vi "UHR-Fleezers Control (host) - 12.0.vi"() -> ()   [LabVIEW 2014] (continued)
        n1231 = Divide(x=w1676, y="APD Integration Time (s)") -> (x/y=w1679:dbl)
        n1232 = Multiply(x=2.0, y=w1679) -> (x*y=w1678:dbl)
        n1233 = local write "APD Samples/FIFO Acq."(w1679) -> ()
        n1234 = local write "APD Elements/DMA read"(w1678) -> ()
      }
      event "Number of F/B Scans (AOD)", "Scan Speed (nm/s)", "Scan BD", "Initial D (MHz)", "Step Size (nm)", "Scan Range (nm)", "Wiggle amp 1 (units?)": Value Change {
        w1747 = 123.0  # AOM cal (nm/MHz)
        n1235 = event-data() -> ()  [unwired: 7 out]
        n1236 = local read "BD 1 Frequency 1 (MHz)"() -> (w1730:dbl)
        n1237 = local read "AOM X Cal (nm/MHz)"() -> (w1722:dbl)
        n1238 = local read "BD 2 Frequency 1 (MHz)"() -> (w1736:dbl)
        n1239 = local read "X RF Frequency Limits (MHz)"() -> (w1734:T17)
        n1240 = local read "Y RF Frequency Limits (MHz)"() -> (w1731:T17)
        n1241 = Negate(x="Scan Range (nm)") -> (-x=w1700:dbl)
        n1242 = Divide(x=w1700, y=w1722) -> (x/y=w1704:dbl)
        n1243 = Select(t=w1734, s="Scan BD", f=w1731) -> (s? t:f=w1733:T17)
        n1244 = Select(t=w1730, s="Scan BD", f=w1736) -> (s? t:f=w1735:dbl)
        n1245 = Unbundle By Name(w1733) -> ("Maximum"=w1742:dbl, "Minimum"=w1741:dbl)
        n1246 = Add(x=w1704, y=w1735) -> (x+y=w1739:dbl)
        n1247 = Divide(x=w1700, y="Step Size (nm)") -> (x/y=w1719:dbl)
        n1248 = Divide(x="Step Size (nm)", y=w1722) -> (x/y=w1728:dbl)
        n1249 = Absolute Value(x=w1719) -> (abs(x)=w1703:dbl)
        n1250 = Sign(1:w1700) -> (0:w1701:dbl)
        n1251 = In Range and Coerce(upper limit=w1742, x=w1739, lower limit=w1741) -> (coerced(x)=w1738:dbl, In Range?=w1740:bool)
        n1252 = To Unsigned Quad Integer(1:w1703) -> (0:w1718:u64)
        "Scan steps (AOD)" <- w1718
        n1253 = call "IR AOM freq to word.vi"("Frequency In (MHz)"=w1728) -> ("Frequency Word Out (double)"=w1725:dbl)
        n1254 = Multiply(x=w1701, y=w1725) -> (x*y=w1702:dbl)
        n1255 = Subtract(x=w1739, y=w1738) -> (x-y=w1737:dbl)
        n1256 = To Quad Integer(1:w1702) -> (0:w1724:i64)
        "Incr. int (AOD)" <- w1724
        n1257 = Subtract(x=w1704, y=w1737) -> (x-y=w1723:dbl)
        "Scan Range (MHz)" <- w1723
        n1258 = Select(t=w1704, s=w1740, f=w1723) -> (s? t:f=w1743:dbl)
        n1259 = Multiply(x=w1723, y=w1722) -> (x*y=w1721:dbl)
        n1260 = Decrement(x=w1718) -> (x-1=w1771:u64)
        n1261 = Negate(x=w1721) -> (-x=w1717:dbl)
        n1262 = local write "Scan Range (nm)"(w1717) -> ()
        n1263 = Divide(x=w1743, y=w1771) -> (x/y=w1727:dbl)
        "Scan Increment (MHz)" <- w1727
        n1264 = call "IR AOM freq to word.vi"("Frequency In (MHz)"=w1727) -> ("Frequency Word Out (double)"=w1726:dbl)
        n1265 = Divide(x="Step Size (nm)", y="Scan Speed (nm/s)") -> (x/y=w1714:dbl)
        n1266 = To Quad Integer(1:w1726) -> ()  [unwired: 1 out]
        n1267 = local read "Number Interlace Sets"() -> (w1698:u8)
        n1268 = local read "AI Count (ticks)"() -> (w1699:u32)
        n1269 = local read "Total Counts (ticks)"() -> (w1697:u32)
        n1270 = local read "# Samples/trap"() -> (w1729:u32)
        n1271 = Multiply(x=w1699, y=w1698) -> (x*y=w1696:u32)
        n1272 = Divide(x=w1697, y=w1696) -> (x/y=w1695:dbl)
        n1273 = Select(t=w1730, s="Scan BD", f=w1736) -> (s? t:f=w1768:dbl)
        "Initial freq. (MHz)" <- w1768
        n1274 = Add(x=w1743, y=w1768) -> (x+y=→"Final freq. (MHz)":dbl)
        n1275 = Divide(x=w1697, y=40000000.0) -> (x/y=w1713:dbl)
        n1276 = Divide(x=w1714, y=w1713) -> (x/y=w1712:dbl)
        n1277 = To Unsigned Quad Integer(1:w1712) -> (0:w1687:u64)
        n1278 = Quotient & Remainder(x=w1687, y=u64 2) -> (x-y*floor(x/y)=w1691:u64)  [unwired: 1 out]
        n1279 = Equal?(x=w1691, y=u64 0) -> (x = y?=w1689:bool)
        n1280 = Decrement(x=w1687) -> (x-1=w1688:u64)
        n1281 = Select(t=w1687, s=w1689, f=w1688) -> (s? t:f=w1686:u64)
        "Cycles/step (AOD)" <- w1686
        n1282 = xnode "Read/Write Control"("FPGA VI Reference In"=w1779, "error in"=w1778, "Scan steps"=w1718, "Number of scans"="Number of F/B Scans (AOD)", "Cycles per step"=w1686, "Scan freq.  increment"=w1724, "Scan BD"="Scan BD") -> ("error out"=w1777:errorcluster)  [unwired: 1 out]
        n1283 = Multiply(x=w1718, y=w1686) -> (x*y=w1772:u64)
        n1284 = Multiply(x=w1772, y=u64 2) -> (x*y=w1694:u64)
        n1285 = Multiply(x=w1695, y=w1694) -> (x*y=w1693:dbl)
        "Data points/scan (f/b)" <- w1693
        n1286 = Multiply(x=w1693, y="Number of F/B Scans (AOD)") -> (x*y=w1775:dbl)
        "Data points/scans" <- w1775
        n1287 = Divide(x=w1775, y=w1729) -> (x/y=→"N sets should be saved":dbl)
        n1288 = Multiply(x=w1772, y=w1713) -> (x*y=w1711:dbl)
        "Time/Scan (s) (AOD)" <- w1711
        n1289 = Select(t=w1743, s="Scan BD", f=0.0) -> (s? t:f=w1769:dbl)
        n1290 = Select(t=0.0, s="Scan BD", f=w1743) -> (s? t:f=w1765:dbl)
        n1291 = local read "BD 2 Frequency 2 (MHz)"() -> (w1761:dbl)
        n1292 = local read "BD 1 Frequency 2 (MHz)"() -> (w1764:dbl)
        n1293 = Add(x=w1765, y=w1736) -> (x+y=w1762:dbl)
        n1294 = Add(x=w1730, y=w1769) -> (x+y=w1763:dbl)
        n1295 = Multiply(x=w1711, y=2.0) -> (x*y=w1710:dbl)
        n1296 = Multiply(x=w1710, y="Number of F/B Scans (AOD)") -> (x*y=w1707:dbl)
        n1297 = Divide(x=w1707, y=60.0) -> (x/y=→"Time to Finish All (min)":dbl)
        n1298 = Add(x="Trap 2 Bead Size (nm)", y="Trap 1 Bead Size (nm)") -> (x+y=w1751:dbl)
        n1299 = Divide(x=w1751, y=2.0) -> (x/y=w1745:dbl)
        n1300 = Subtract(x=w1762, y=w1761) -> (x-y=w1759:dbl)
        n1301 = Subtract(x=w1763, y=w1764) -> (x-y=w1760:dbl)
        n1302 = local read "Initial D (MHz)"() -> (w1748:dbl)
        n1303 = Square(x=w1759) -> (x^2=w1758:dbl)
        n1304 = Square(x=w1760) -> (x^2=w1757:dbl)
        n1305 = Add(x=w1757, y=w1758) -> (x+y=w1756:dbl)
        n1306 = Square Root(x=w1756) -> (sqrt(x)=w1755:dbl)
        "Final D (MHz)" <- w1755
        n1307 = Multiply(x=w1747, y=w1755) -> (x*y=w1754:dbl)
        n1308 = Multiply(x=w1748, y=w1747) -> (x*y=w1746:dbl)
        n1309 = Subtract(x=w1746, y=w1745) -> (x-y=→"Initial sep (nm)":dbl)
        n1310 = Subtract(x=w1754, y=w1745) -> (x-y=→"Final sep (nm)":dbl)
      }
      event "Freq or Amp switch first", "Swap F1 and F2", "Freq switch delay", "Amp switch delay": Value Change {
        n1311 = event-data() -> ()  [unwired: 7 out]
        n1312 = local read "Freq or Amp switch first"() -> (w1780:bool)
        n1313 = local read "Amp switch delay"() -> (w1781:u16)
        n1314 = local read "Freq switch delay"() -> (w1783:u16)
        n1315 = local read "Swap F1 and F2"() -> (w1782:bool)
        n1316 = xnode "Read/Write Control"("FPGA VI Reference In"=w1786, "error in"=w1785, "Freq switch delay"=w1783, "Swap F1 and F2"=w1782, "Amp switch delay"=w1781, "Freq or Amp switch first"=w1780) -> ("error out"=w1784:errorcluster)  [unwired: 1 out]
      }
      event "Scan steps (MCL)", "Number of scans (MCL)", "Scan Range (V)\n(of steps)", "2D or 1D Scan", "N APD Samp/step", "Fast Scan Dir", "Continuous MCL Scanning", "Scan lines (y)": Value Change {
        w1788 = 32767.0 ("y")
        n1317 = event-data() -> ()  [unwired: 7 out]
        n1318 = Select(t="Scan lines (y)", s="2D or 1D Scan", f="Number of scans (MCL)") -> (s? t:f=w1793:u64)
        n1319 = Decrement(x="Scan steps (MCL)") -> (x-1=w1809:u64)
        n1320 = Divide(x="Scan Range (V)\n(of steps)", y=w1809) -> (x/y=w1808:dbl)
        "Desired Scan Incr (V)" <- w1808
        n1321 = local read "APD Integration Time (s)"() -> (w1801:dbl)
        n1322 = Multiply(x=w1808, y=w1788) -> (x*y=w1817:dbl)
        n1323 = Divide(x=w1817, y=10.0) -> (x/y=w1807:dbl)
        "Desired incr (int)" <- w1807
        n1324 = local read "Update Count (MCL)"() -> (w1813:u32)
        n1325 = Round Toward -Infinity(1:w1807) -> (0:w1816:dbl)
        n1326 = To Word Integer(number=w1816) -> (16bit integer=w1791:i16)
        "Actual Incr. int (MCL)" <- w1791
        n1327 = Multiply(x=w1801, y=40000000.0) -> (x*y=w1814:dbl)
        n1328 = Divide(x=w1814, y=w1813) -> (x/y=w1812:dbl)
        n1329 = Multiply(x=i16 10, y=w1791) -> (x*y=w1789:i16)
        n1330 = Multiply(x="N APD Samp/step", y=w1812) -> (x*y=w1811:dbl)
        "Cycles/step (MCL)" <- w1811
        n1331 = Divide(x=w1789, y=w1788) -> (x/y=→"Actual MCL Inc (V)":dbl)
        n1332 = Multiply(x="N APD Samp/step", y="Scan steps (MCL)") -> (x*y=w1803:dbl)
        n1333 = local read "APD Samples/FIFO Acq."() -> (w1800:dbl)
        n1334 = Multiply(x=w1803, y=u64 2) -> (x*y=w1802:dbl)
        "Data points/scan (f+b)" <- w1802
        n1335 = Multiply(x=w1802, y=w1793) -> (x*y=w1820:dbl)
        "Data points/scans (MCL)" <- w1820
        n1336 = Multiply(x=w1801, y=w1802) -> (x*y=w1794:dbl)
        "Time/f+b scan (s) (MCL)" <- w1794
        n1337 = Divide(x=w1820, y=w1800) -> (x/y=→"N sets should be saved (MCL)":dbl)
        n1338 = Multiply(x=w1794, y=w1793) -> (x*y=→"Total Time (s)":dbl)
        n1339 = Not(x="Fast Scan Dir") -> (.not. x?=w1798:bool)
        n1340 = xnode "Read/Write Control"("FPGA VI Reference In"=w1824, "error in"=w1823, "Scan steps (MCL)"="Scan steps (MCL)", "Number of scans (MCL)"=w1793, "Cycles per step (MCL)"=w1811, "Scan freq.  increment (MCL)"=w1791, "1D or 2D Scan?"="2D or 1D Scan", "MCL Scan Axis"=w1798, "Cont. Scan (MCL)"="Continuous MCL Scanning") -> ("error out"=w1822:errorcluster)  [unwired: 1 out]
      }
      event "Read Cal": Value Change {
        w1826 = 1000.0 ("y")
        n1341 = event-data() -> ()  [unwired: 7 out]
        n1342 = local read "Save file name"() -> (w1851:path)
        n1343 = local write "Read Cal"(FALSE ("Read Cal")) -> ()
        n1344 = Strip Path(path=w1851) -> (stripped path=w1850:path)  [unwired: 1 out]
        n1345 = Path To String(path=w1850) -> (string=w1849:string)
        n1346 = Concatenate Strings(w1849, "\\current.cal" ("string")) -> (w1847:string)
        n1347 = String To Path(string=w1847) -> (path=w1846:path)
        n1348 = Open/Create/Replace File(file path (use dialog)=w1846, operation (0:open)=T30."open", access (0:read/write)=enum16{"read/write", "read-only", "write-only"}."read-only") -> (refnum out=w1854:refnum<file>, error out=w1840:errorcluster)  [unwired: 1 in, 3 out]
        n1349 = Deny Access(4:w1840, 7:w1854) -> (0:w1839:errorcluster, 3:w1845:refnum<file>)  [unwired: 1 out]
        n1350 = Read from Binary File(5:0.0, 8:w1839, 9:T29."big-endian, network order" ("byte order (0:big-endian, network order)"), 10:-1 ("count (1)"), 11:w1845) -> (0:w1838:errorcluster, 2:w1836:dbl[], 3:w1841:refnum<file>)  [unwired: 2 out]
        n1351 = Array To Cluster(array=w1836) -> (cluster=w1835:T32)
        n1352 = Unbundle(w1835) -> ("[0]"=w1834:dbl, "[1]"=w1833:dbl, "[2]"=w1832:dbl, "[3]"=w1831:dbl, "[4]"=w1830:dbl, "[5]"=w1829:dbl)
        n1353 = Close File(refnum=w1841, error in=w1838) -> (error out=→"Read cal error":errorcluster)  [unwired: 1 out]
        n1354 = Multiply(x=w1829, y=w1826) -> (x*y=w1827:dbl)
        n1355 = local write "T2 k_x (pN/nm)"(w1831) -> ()
        n1356 = local write "T1 k_x (pN/nm)"(w1832) -> ()
        n1357 = local write "T1 a_x (nm/V)"(w1834) -> ()
        n1358 = local write "T2 a_x (nm/V)"(w1833) -> ()
        n1359 = Multiply(x=w1830, y=w1826) -> (x*y=w1828:dbl)
        n1360 = local write "T1 offset_x (mV)"(w1828) -> ()
        n1361 = local write "T2 offset_x (mV)"(w1827) -> ()
      }
      event "Read FX file": Value Change {
        n1362 = event-data() -> ()  [unwired: 7 out]
        n1363 = local write "Read FX file"(FALSE ("Read residual")) -> ()
        n1364 = local read "Save file name"() -> (w1879:path)
        n1365 = Strip Path(path=w1879) -> (stripped path=w1878:path)  [unwired: 1 out]
        n1366 = Path To String(path=w1878) -> (string=w1877:string)
        n1367 = Concatenate Strings(w1877, "\\current.cal" ("string")) -> (w1875:string)
        n1368 = String To Path(string=w1875) -> (path=w1874:path)
        n1369 = Open/Create/Replace File(file path (use dialog)=w1874, operation (0:open)=T30."open", access (0:read/write)=enum16{"read/write", "read-only", "write-only"}."read-only") -> (refnum out=w1871:refnum<file>, error out=w1868:errorcluster)  [unwired: 3 in, 1 out]
        n1370 = Deny Access(4:w1868, 7:w1871) -> (0:w1867:errorcluster, 3:w1870:refnum<file>)  [unwired: 1 in]
        n1371 = Read from Binary File(5:0.0, 8:w1867, 9:T29."big-endian, network order" ("byte order (0:big-endian, network order)"), 10:-1 ("count"), 11:w1870) -> (0:w1863:errorcluster, 2:w1857:dbl[], 3:w1864:refnum<file>)  [unwired: 1 in, 1 out]
        n1372 = Index Array(array=w1857, index=6) -> (element=→"Bad fit error":dbl)
        n1373 = Index Array(array=w1857, index=7) -> (element=→"Fit offset":dbl)
        n1374 = Index Array(array=w1857, index=8) -> (element=→"Hyst. error":dbl)
        n1375 = Close File(refnum=w1864, error in=w1863) -> ()  [unwired: 2 out]
      }
      event "Abort MCL Scan": Value Change {
        n1376 = event-data() -> ()  [unwired: 7 out]
        n1377 = local write "MCL Scanning"(FALSE ("MCL Scanning")) -> ()
        n1378 = xnode "Read/Write Control"("FPGA VI Reference In"=w1884, "error in"=w1883, "Abort scan (MCL)"="Abort MCL Scan") -> ("error out"=w1882:errorcluster)  [unwired: 1 out]
      }
      event "Update Count (MCL)": Value Change {
        n1379 = event-data() -> ()  [unwired: 7 out]
        n1380 = xnode "Read/Write Control"("FPGA VI Reference In"=w1888, "error in"=w1887, "MCL count"="Update Count (MCL)") -> ("error out"=w1886:errorcluster)  [unwired: 1 out]
      }
      event "Phase adjust (MCL)", "+ phase (MCL)", "- phase (MCL)": Value Change {
        n1381 = event-data() -> ()  [unwired: 7 out]
        n1382 = Negate(x="Phase adjust (MCL)") -> (-x=w1897:i16)
        n1383 = Select(t=w1897, s="- phase (MCL)", f="Phase adjust (MCL)") -> (s? t:f=w1895:i16)
        n1384 = Or(x="- phase (MCL)", y="+ phase (MCL)") -> (x .or. y?=w1890:bool)
        n1385 = xnode "Read/Write Control"("FPGA VI Reference In"=w1899, "error in"=w1898, "Phase count adjustment (MCL)"=w1895) -> ("FPGA VI Reference Out"=w1891:T22, "error out"=w1892:errorcluster)
        n1386 = xnode "Read/Write Control"("FPGA VI Reference In"=w1891, "error in"=w1892, "+ phase (MCL)"=w1890) -> ("error out"=w1889:errorcluster)  [unwired: 1 out]
      }
      event "Abort AOD Scan": Value Change {
        n1387 = event-data() -> ()  [unwired: 7 out]
        n1388 = xnode "Read/Write Control"("FPGA VI Reference In"=w1903, "error in"=w1902, "Abort scan"="Abort AOD Scan") -> ("error out"=w1901:errorcluster)  [unwired: 1 out]
      }
      event "Continuous AOD Scanning": Value Change {
        n1389 = event-data() -> ()  [unwired: 7 out]
        n1390 = xnode "Read/Write Control"("FPGA VI Reference In"=w1907, "error in"=w1906, "Cont. Scan"="Continuous AOD Scanning") -> ("error out"=w1905:errorcluster)  [unwired: 1 out]
      }
      event "Index": Value Change {
        n1391 = event-data() -> ()  [unwired: 7 out]
        n1392 = call "Create new save file.vi"("Insert"="", "Ext"=".dat" ("string"), "Index In"="Index") -> ("Path Out"=→"Save file name":path, "Index Out"=w1908:dbl)
        "Save index" <- w1908
        n1393 = local write "Index"(w1908) -> ()
      }
      event "AO1", "AO2": Value Change {
        w1923 = 10.0 ("y")
        w1922 = 32767.0 ("y")
        n1394 = event-data() -> ()  [unwired: 7 out]
        n1395 = local read "AO2"() -> (w1921:dbl)
        n1396 = local read "AO1"() -> (w1918:dbl)
        n1397 = Multiply(x=w1918, y=w1922) -> (x*y=w1917:dbl)
        n1398 = Multiply(x=w1921, y=w1922) -> (x*y=w1920:dbl)
        n1399 = Divide(x=w1917, y=w1923) -> (x/y=w1916:dbl)
        n1400 = Divide(x=w1920, y=w1923) -> (x/y=w1919:dbl)
        n1401 = To Word Integer(number=w1916) -> (16bit integer=w1924:i16)
        n1402 = To Word Integer(number=w1919) -> (16bit integer=w1925:i16)
        n1403 = xnode "Read/Write Control"("FPGA VI Reference In"=w1915, "error in"=w1914, "AO1"=w1924, "AO2"=w1925) -> ("error out"=w1913:errorcluster)  [unwired: 1 out]
      }
      event "Inject Pump 1": Value Change {
        n1404 = event-data() -> ()  [unwired: 7 out]
        n1405 = local read "Use Harvard pumps\nfor beads (else Chemyx)"() -> (w1927:bool)
        n1406 = case shown="True" w1927 {
          tunnel: "Inject Pump 1" -> [w1931 w1969]
          tunnel: w1926 -> [_ w1970]
          frame False {
            n1407 = local read "Pump write delay (ms)"() -> (w1930:dbl)
            n1408 = local read "Chemyx Syringe Pump Serial Port"() -> (w1929:refnum<visa-resource-name>)
            n1409 = case shown="True" w1931 {
              tunnel: w1930 -> [w1937 w1951]
              tunnel: w1929 -> [w1934 w1950]
              frame False {
                n1410 = flat-sequence {
                  tunnel: w1934 -> [w1938]
                  tunnel: [w1938] -> w1935
                  tunnel: w1937 -> [_]
                  tunnel: [w1941] -> w1936
                  tunnel: w1935 -> [w1941]
                  tunnel: w1936 -> [w1942]
                  tunnel: [w1942] -> w1932
                  tunnel: [w1944] -> w1933
                  tunnel: w1932 -> [w1944]
                  tunnel: w1933 -> [w1946]
                  frame #0 {
                    n1411 = call "Write to pump.vi"("string"="enter pump1", "VISA resource name"=w1938) -> ()  [unwired: 1 out]
                  }
                  frame #1 {
                    n1412 = Wait (ms)(milliseconds to wait="Pump pause delay (ms)") -> ()  [unwired: 1 out]
                  }
                  frame #2 {
                    n1413 = call "Write to pump.vi"("string"="stop", "VISA resource name"=w1942) -> ()  [unwired: 1 out]
                  }
                  frame #3 {
                    n1414 = Wait (ms)(milliseconds to wait=u32 500) -> ()  [unwired: 1 out]
                  }
                  frame #4 {
                    n1415 = call "Write to pump.vi"("string"="stop", "VISA resource name"=w1946) -> ()  [unwired: 1 out]
                  }
                }
              }
              frame True {
                n1416 = flat-sequence {
                  tunnel: w1950 -> [w1960]
                  tunnel: w1951 -> [w1955]
                  tunnel: w1951 -> [w1962]
                  tunnel: w1950 -> [w1963]
                  tunnel: [w1963] -> w1948
                  tunnel: [w1965] -> w1949
                  tunnel: w1948 -> [w1965]
                  tunnel: w1949 -> [w1967]
                  frame #0 {
                    n1417 = local read "All Pump Parameters"() -> (w1954:T5)
                    n1418 = Unbundle By Name(w1954) -> ("Pump 1"=w1961:T33)
                    n1419 = call "Set pump parameters.vi"("Pump write delay (ms)"=w1955, "Volume (uL)"="Ch 1 Inject Volume (uL)", "Rate (uL/h)"="Ch 1 Inject Rate (ul/h)", "Units"=4.0, "Pump #"=1.0, "Pump Parameters In"=w1961, "VISA resource name"=w1960) -> ("Pump Parameters Out"=w1953:T33)  [unwired: 3 in]
                    n1420 = Bundle By Name(cluster=w1954, "Pump 1"=w1953) -> (w1952:T5)
                    n1421 = local write "All Pump Parameters"(w1952) -> ()
                  }
                  frame #1 {
                    n1422 = Wait (ms)(milliseconds to wait=w1962) -> ()  [unwired: 1 out]
                  }
                  frame #2 {
                    n1423 = call "Write to pump.vi"("string"="start", "VISA resource name"=w1963) -> ()  [unwired: 1 out]
                  }
                  frame #3 {
                    n1424 = Wait (ms)(milliseconds to wait=u32 500) -> ()  [unwired: 1 out]
                  }
                  frame #4 {
                    n1425 = call "Write to pump.vi"("string"="start", "VISA resource name"=w1967) -> ()  [unwired: 1 out]
                  }
                }
              }
            }
          }
          frame True {
            n1426 = case shown="True" w1969 {
              tunnel: w1970 -> [w1971 w1981]
              frame False {
                n1427 = flat-sequence {
                  tunnel: w1971 -> [w1973]
                  frame #0 {
                    n1428 = local write "Flushing P1"(FALSE ("Flushing P1")) -> ()
                    n1429 = Concatenate Strings("stop" ("string"), "\r") -> (w1975:string)
                    n1430 = VISA Write(VISA resource name=w1973, write buffer=w1975) -> ()  [unwired: 1 in, 3 out]
                  }
                  frame #1 {
                    n1431 = property on="Clear Volume P1" class="Bool (strict)"("Val(Sgnl)"=TRUE ("Value (Signaling)")) -> ()  [unwired: 2 in, 2 out]
                  }
                }
              }
              frame True {
                n1432 = local read "Normal Flow Rate (ul/h) P1"() -> (w1979:dbl)
                n1433 = Number To Decimal String(number=w1979) -> (decimal integer string=w1985:string)  [unwired: 1 in]
                n1434 = Concatenate Strings("irate  " ("string"), w1985, " u/h" ("string"), "\r") -> (w1983:string)
                n1435 = VISA Write(VISA resource name=w1981, write buffer=w1983) -> (VISA resource name out=w1980:refnum<visa-resource-name>)  [unwired: 1 in, 2 out]
                n1436 = Concatenate Strings("irun" ("string"), "\r") -> (w1987:string)
                n1437 = VISA Write(VISA resource name=w1980, write buffer=w1987) -> ()  [unwired: 1 in, 3 out]
              }
            }
          }
        }
      }
      event "Inject Pump 3": Value Change {
        n1438 = event-data() -> ()  [unwired: 7 out]
        n1439 = local read "Use Harvard pumps\nfor beads (else Chemyx)"() -> (w1990:bool)
        n1440 = case shown="True" w1990 {
          tunnel: "Inject Pump 3" -> [w1994 w2033]
          tunnel: w1989 -> [_ w2032]
          frame False {
            n1441 = local read "Pump write delay (ms)"() -> (w1993:dbl)
            n1442 = case shown="True" w1994 {
              tunnel: w1993 -> [w2000 w2014]
              tunnel: "Chemyx Syringe Pump Serial Port" -> [w1997 w2013]
              frame False {
                n1443 = flat-sequence {
                  tunnel: w1997 -> [w2001]
                  tunnel: [w2001] -> w1998
                  tunnel: w2000 -> [_]
                  tunnel: [w2004] -> w1999
                  tunnel: w1998 -> [w2004]
                  tunnel: w1999 -> [w2005]
                  tunnel: [w2005] -> w1995
                  tunnel: [w2007] -> w1996
                  tunnel: w1995 -> [w2007]
                  tunnel: w1996 -> [w2009]
                  frame #0 {
                    n1444 = call "Write to pump.vi"("string"="enter pump3", "VISA resource name"=w2001) -> ()  [unwired: 1 out]
                  }
                  frame #1 {
                    n1445 = local read "Pump pause delay (ms)"() -> (w2003:u32)
                    n1446 = Wait (ms)(milliseconds to wait=w2003) -> ()  [unwired: 1 out]
                  }
                  frame #2 {
                    n1447 = call "Write to pump.vi"("string"="stop", "VISA resource name"=w2005) -> ()  [unwired: 1 out]
                  }
                  frame #3 {
                    n1448 = Wait (ms)(milliseconds to wait=u32 0) -> ()  [unwired: 1 out]
                  }
                  frame #4 {
                    n1449 = call "Write to pump.vi"("string"="stop", "VISA resource name"=w2009) -> ()  [unwired: 1 out]
                  }
                }
              }
              frame True {
                n1450 = flat-sequence {
                  tunnel: w2013 -> [w2023]
                  tunnel: w2014 -> [w2018]
                  tunnel: w2014 -> [w2025]
                  tunnel: w2013 -> [w2026]
                  tunnel: [w2026] -> w2012
                  tunnel: [w2029] -> w2011
                  tunnel: w2012 -> [w2029]
                  tunnel: w2011 -> [w2030]
                  frame #0 {
                    n1451 = local read "All Pump Parameters"() -> (w2017:T5)
                    n1452 = Unbundle By Name(w2017) -> ("Pump 3"=w2024:T33)
                    n1453 = call "Set pump parameters.vi"("Pump write delay (ms)"=w2018, "Volume (uL)"="Ch 3 Inject Volume (uL)", "Rate (uL/h)"="Ch 3 Inject Rate (ul/h)", "Units"=4.0, "Pump #"=3.0, "Pump Parameters In"=w2024, "VISA resource name"=w2023) -> ("Pump Parameters Out"=w2016:T33)  [unwired: 3 in]
                    n1454 = Bundle By Name(cluster=w2017, "Pump 3"=w2016) -> (w2015:T5)
                    n1455 = local write "All Pump Parameters"(w2015) -> ()
                  }
                  frame #1 {
                    n1456 = Wait (ms)(milliseconds to wait=w2025) -> ()  [unwired: 1 out]
                  }
                  frame #2 {
                    n1457 = call "Write to pump.vi"("string"="start", "VISA resource name"=w2026) -> ()  [unwired: 1 out]
                  }
                  frame #3 {
                    n1458 = Wait (ms)(milliseconds to wait=u32 500) -> ()  [unwired: 1 out]
                  }
                  frame #4 {
                    n1459 = call "Write to pump.vi"("string"="start", "VISA resource name"=w2030) -> ()  [unwired: 1 out]
                  }
                }
              }
            }
          }
          frame True {
            n1460 = case shown="True" w2033 {
              tunnel: w2032 -> [w2034 w2041]
              frame False {
                n1461 = flat-sequence {
                  tunnel: w2034 -> [w2036]
                  frame #0 {
                    n1462 = local write "Flushing P3"(FALSE ("Flushing P3")) -> ()
                    n1463 = Concatenate Strings("stop" ("string"), "\r") -> (w2038:string)
                    n1464 = VISA Write(VISA resource name=w2036, write buffer=w2038) -> ()  [unwired: 1 in, 3 out]
                  }
                  frame #1 {
                    n1465 = property on="Clear Volume P3" class="Bool (strict)"("Val(Sgnl)"=TRUE ("Value (Signaling)")) -> ()  [unwired: 2 in, 2 out]
                  }
                }
              }
              frame True {
                n1466 = local read "Normal Flow Rate (ul/h) P3"() -> (w2042:dbl)
                n1467 = Number To Decimal String(number=w2042) -> (decimal integer string=w2048:string)  [unwired: 1 in]
                n1468 = Concatenate Strings("irate  " ("string"), w2048, " u/h" ("string"), "\r") -> (w2046:string)
                n1469 = VISA Write(VISA resource name=w2041, write buffer=w2046) -> (VISA resource name out=w2044:refnum<visa-resource-name>)  [unwired: 1 in, 2 out]
                n1470 = Concatenate Strings("irun" ("string"), "\r") -> (w2050:string)
                n1471 = VISA Write(VISA resource name=w2044, write buffer=w2050) -> ()  [unwired: 1 in, 3 out]
              }
            }
          }
        }
      }
      event "Inject Pump 2": Value Change {
        n1472 = event-data() -> ()  [unwired: 7 out]
        n1473 = local read "Pump write delay (ms)"() -> (w2054:dbl)
        n1474 = local read "Chemyx Syringe Pump Serial Port"() -> (w2052:refnum<visa-resource-name>)
        n1475 = flat-sequence {
          tunnel: w2052 -> [w2067]
          tunnel: w2054 -> [w2063]
          tunnel: "Inject Pump 2" -> [_]
          tunnel: w2054 -> [w2069]
          tunnel: w2052 -> [w2070]
          frame #0 {
            n1476 = local read "All Pump Parameters"() -> (w2062:T5)
            n1477 = Multiply(x=60.0, y="Flush Center Ch Rate (ul/m)") -> (x*y=w2059:dbl)
            n1478 = Unbundle By Name(w2062) -> ("Pump 2"=w2068:T33)
            n1479 = call "Set pump parameters.vi"("Pump write delay (ms)"=w2063, "Volume (uL)"="Flush Center Ch Volume (uL)", "Rate (uL/h)"=w2059, "Units"=3.0, "Pump #"=2.0, "Pump Parameters In"=w2068, "VISA resource name"=w2067) -> ("Pump Parameters Out"=w2061:T33)  [unwired: 3 in]
            n1480 = Bundle By Name(cluster=w2062, "Pump 2"=w2061) -> (w2060:T5)
            n1481 = Add(x="Flush Center Ch Volume (uL)", y="Total Volume\nFlushed (uL)") -> (x+y=w2056:dbl)
            n1482 = local write "All Pump Parameters"(w2060) -> ()
            n1483 = local write "Total Volume\nFlushed (uL)"(w2056) -> ()
          }
          frame #1 {
            n1484 = Wait (ms)(milliseconds to wait=w2069) -> ()  [unwired: 1 out]
          }
          frame #2 {
            n1485 = call "Write to pump.vi"("string"="start", "VISA resource name"=w2070) -> ()  [unwired: 1 out]
          }
        }
      }
      event "Sample Channel\nFlow": Value Change {
        n1486 = event-data() -> ()  [unwired: 7 out]
        n1487 = case shown="True" "Sample Channel\nFlow" {
          tunnel: w2073 -> [w2074 w2080]
          frame False {
            n1488 = flat-sequence {
              tunnel: w2074 -> [w2076]
              frame #0 {
                n1489 = local write "Flushing samp"(FALSE ("Flushing samp")) -> ()
                n1490 = Concatenate Strings("stop" ("string"), "\r") -> (w2079:string)
                n1491 = VISA Write(VISA resource name=w2076, write buffer=w2079) -> ()  [unwired: 1 in, 3 out]
              }
            }
          }
          frame True {
            n1492 = local read "Normal Flow rate (mL/h)"() -> (w2090:dbl)
            n1493 = Number To Decimal String(number=w2090) -> (decimal integer string=w2089:string)  [unwired: 1 in]
            n1494 = Concatenate Strings("irate " ("string"), w2089, " u/h" ("string"), "\r") -> (w2085:string)
            n1495 = VISA Write(VISA resource name=w2080, write buffer=w2085) -> (VISA resource name out=w2084:refnum<visa-resource-name>)  [unwired: 1 in, 2 out]
            n1496 = Concatenate Strings("irun" ("string"), "\r") -> (w2081:string)
            n1497 = VISA Write(VISA resource name=w2084, write buffer=w2081) -> ()  [unwired: 1 in, 3 out]
          }
        }
      }
      event "Start Flow": Value Change {
        n1498 = event-data() -> ()  [unwired: 7 out]
        n1499 = local write "Sample Channel\nFlow"(TRUE ("Sample Channel\nFlow")) -> ()
        n1500 = local write "Start Flow"(FALSE ("Start Flow")) -> ()
        n1501 = Concatenate Strings("irun" ("string"), "\r") -> (w2095:string)
        n1502 = VISA Write(VISA resource name=w2091, write buffer=w2095) -> ()  [unwired: 1 in, 3 out]
      }
      event "Stop Flow": Value Change {
        w2097 = FALSE ("Stop Flow")
        n1503 = event-data() -> ()  [unwired: 7 out]
        n1504 = local write "Stop Flow"(w2097) -> ()
        n1505 = local write "Sample Channel\nFlow"(w2097) -> ()
        n1506 = Concatenate Strings("stop" ("string"), "\r") -> (w2100:string)
        n1507 = VISA Write(VISA resource name=w2098, write buffer=w2100) -> ()  [unwired: 1 in, 3 out]
      }
      event "Normal Flow rate (mL/h)": Value Change {
        n1508 = event-data() -> ()  [unwired: 7 out]
        n1509 = Number To Decimal String(number="Normal Flow rate (mL/h)") -> (decimal integer string=w2107:string)  [unwired: 1 in]
        n1510 = Concatenate Strings("irate  " ("string"), w2107, " u/h" ("string"), "\r") -> (w2106:string)
        n1511 = VISA Write(VISA resource name=w2103, write buffer=w2106) -> ()  [unwired: 1 in, 3 out]
      }
      event "Flush Sample": Value Change {
        n1512 = event-data() -> ()  [unwired: 7 out]
        n1513 = flat-sequence {
          tunnel: w2109 -> [w2137]
          frame #0 {
            # "set parameters (rate, volume) for flush, clear volume"
            n1514 = Number To Decimal String(number="Flush rate (mL/m)") -> (decimal integer string=w2133:string)  [unwired: 1 in]
            n1515 = local write "Sample Channel\nFlow"(TRUE ("Sample Channel\nFlow")) -> ()
            n1516 = Concatenate Strings("irate  " ("string"), w2133, " u/m" ("string"), "\r") -> (w2135:string)
            n1517 = VISA Write(VISA resource name=w2137, write buffer=w2135) -> (VISA resource name out=w2131:refnum<visa-resource-name>)  [unwired: 1 in, 2 out]
            n1518 = Number To Decimal String(number="Flush volume (mL)") -> (decimal integer string=w2122:string)  [unwired: 1 in]
            n1519 = Reciprocal(x="Flush rate (mL/m)") -> (1/x=w2116:dbl)
            n1520 = Concatenate Strings("tvolume  " ("string"), w2122, " u" ("string"), "\r") -> (w2120:string)
            n1521 = Multiply(x=w2116, y="Flush volume (mL)") -> (x*y=w2114:dbl)
            n1522 = VISA Write(VISA resource name=w2131, write buffer=w2120) -> (VISA resource name out=w2119:refnum<visa-resource-name>)  [unwired: 1 in, 2 out]
            n1523 = Multiply(x=w2114, y=60.0) -> (x*y=→"Samp Flush Time (s)":dbl)
            n1524 = Concatenate Strings("cvolume" ("string"), "\r") -> (w2118:string)
            n1525 = VISA Write(VISA resource name=w2119, write buffer=w2118) -> (VISA resource name out=w2129:refnum<visa-resource-name>)  [unwired: 1 in, 2 out]
            n1526 = Concatenate Strings("irun" ("string"), "\r") -> (w2127:string)
            n1527 = VISA Write(VISA resource name=w2129, write buffer=w2127) -> ()  [unwired: 1 in, 3 out]
          }
          frame #1 {
            "Flushing samp" <- TRUE ("Boolean")
          }
        }
      }
      event "Flush Pump 3": Value Change {
        n1528 = event-data() -> ()  [unwired: 7 out]
        n1529 = flat-sequence {
          tunnel: w2139 -> [w2142]
          frame #0 {
            # "set paramaters (rate, volume) for flush, clear volume"
            n1530 = Number To Decimal String(number="Flush rate (uL/m) P3") -> (decimal integer string=w2164:string)  [unwired: 1 in]
            n1531 = local write "Inject Pump 3"(TRUE ("Inject Pump 3")) -> ()
            n1532 = Concatenate Strings("irate  " ("string"), w2164, " u/m" ("string"), "\r") -> (w2166:string)
            n1533 = VISA Write(VISA resource name=w2142, write buffer=w2166) -> (VISA resource name out=w2162:refnum<visa-resource-name>)  [unwired: 1 in, 2 out]
            n1534 = Reciprocal(x="Flush rate (uL/m) P3") -> (1/x=w2146:dbl)
            n1535 = Number To Decimal String(number="Volume (uL) P3") -> (decimal integer string=w2153:string)  [unwired: 1 in]
            n1536 = Multiply(x="Volume (uL) P3", y=w2146) -> (x*y=w2145:dbl)
            n1537 = Concatenate Strings("tvolume  " ("string"), w2153, " u" ("string"), "\r") -> (w2151:string)
            n1538 = Multiply(x=w2145, y=60.0) -> (x*y=→"HP3 Flush Time (s)":dbl)
            n1539 = VISA Write(VISA resource name=w2162, write buffer=w2151) -> (VISA resource name out=w2150:refnum<visa-resource-name>)  [unwired: 1 in, 2 out]
            n1540 = Concatenate Strings("cvolume" ("string"), "\r") -> (w2149:string)
            n1541 = VISA Write(VISA resource name=w2150, write buffer=w2149) -> (VISA resource name out=w2160:refnum<visa-resource-name>)  [unwired: 1 in, 2 out]
            n1542 = Concatenate Strings("irun" ("string"), "\r") -> (w2158:string)
            n1543 = VISA Write(VISA resource name=w2160, write buffer=w2158) -> ()  [unwired: 1 in, 3 out]
          }
          frame #1 {
            "Flushing P3" <- TRUE ("Flushing P3")
          }
        }
      }
      event "Flush Pump 1": Value Change {
        n1544 = event-data() -> ()  [unwired: 7 out]
        n1545 = flat-sequence {
          tunnel: [w2180] -> w2170
          tunnel: w2169 -> [w2173]
          tunnel: w2170 -> [_]
          frame #0 {
            # "set paramaters (rate, volume) for flush, clear volume"
            n1546 = local write "Inject Pump 1"(TRUE ("Inject Pump 1")) -> ()
            n1547 = Number To Decimal String(number="Flush rate (uL/m) P1") -> (decimal integer string=w2196:string)  [unwired: 1 in]
            n1548 = Concatenate Strings("irate  " ("string"), w2196, " u/m" ("string"), "\r") -> (w2198:string)
            n1549 = VISA Write(VISA resource name=w2173, write buffer=w2198) -> (VISA resource name out=w2194:refnum<visa-resource-name>)  [unwired: 1 in, 2 out]
            n1550 = Reciprocal(x="Flush rate (uL/m) P1") -> (1/x=w2177:dbl)
            n1551 = Number To Decimal String(number="Volume (uL) P1") -> (decimal integer string=w2185:string)  [unwired: 1 in]
            n1552 = Multiply(x="Volume (uL) P1", y=w2177) -> (x*y=w2176:dbl)
            n1553 = Concatenate Strings("tvolume  " ("string"), w2185, " u" ("string"), "\r") -> (w2183:string)
            n1554 = Multiply(x=w2176, y=60.0) -> (x*y=→"HP1 Flush Time (s)":dbl)
            n1555 = VISA Write(VISA resource name=w2194, write buffer=w2183) -> (VISA resource name out=w2182:refnum<visa-resource-name>)  [unwired: 1 in, 2 out]
            n1556 = Concatenate Strings("cvolume" ("string"), "\r") -> (w2181:string)
            n1557 = VISA Write(VISA resource name=w2182, write buffer=w2181) -> (VISA resource name out=w2192:refnum<visa-resource-name>)  [unwired: 1 in, 2 out]
            n1558 = Concatenate Strings("irun" ("string"), "\r") -> (w2190:string)
            n1559 = VISA Write(VISA resource name=w2192, write buffer=w2190) -> (VISA resource name out=w2180:refnum<visa-resource-name>)  [unwired: 1 in, 2 out]
          }
          frame #1 {
            "Flushing P1" <- TRUE ("Flushing P3")
          }
        }
      }
      event "Clear Volume": Value Change {
        n1560 = event-data() -> ()  [unwired: 7 out]
        n1561 = Number To Decimal String(number="Normal volume (mL)") -> (decimal integer string=w2205:string)  [unwired: 1 in]
        n1562 = Concatenate Strings("tvolume " ("string"), w2205, " u" ("string"), "\r") -> (w2202:string)
        n1563 = VISA Write(VISA resource name=w2208, write buffer=w2202) -> (VISA resource name out=w2201:refnum<visa-resource-name>)  [unwired: 1 in, 2 out]
        n1564 = local write "Clear Volume"(FALSE ("Clear Volume")) -> ()
        n1565 = Concatenate Strings("cvolume" ("string"), "\r") -> (w2210:string)
        n1566 = VISA Write(VISA resource name=w2201, write buffer=w2210) -> ()  [unwired: 1 in, 3 out]
      }
      event "Clear Volume P3": Value Change {
        n1567 = event-data() -> ()  [unwired: 7 out]
        n1568 = Concatenate Strings("cvolume" ("string"), "\r") -> (w2216:string)
        n1569 = VISA Write(VISA resource name=w2215, write buffer=w2216) -> ()  [unwired: 1 in, 3 out]
        n1570 = local write "Clear Volume P3"(FALSE ("Clear Volume P3")) -> ()
      }
      event "Clear Volume P1": Value Change {
        n1571 = event-data() -> ()  [unwired: 7 out]
        n1572 = Concatenate Strings("cvolume" ("string"), "\r") -> (w2221:string)
        n1573 = local write "Clear Volume P1"(FALSE ("Clear Volume P1")) -> ()
        n1574 = VISA Write(VISA resource name=w2220, write buffer=w2221) -> ()  [unwired: 1 in, 3 out]
      }
      event "Display On P3": Value Change {
        n1575 = event-data() -> ()  [unwired: 7 out]
        n1576 = Select(t="dim 100", s="Display On P3", f="dim 0") -> (s? t:f=w2227:string)
        n1577 = Concatenate Strings(w2227, "\r") -> (w2229:string)
        n1578 = VISA Write(VISA resource name=w2224, write buffer=w2229) -> ()  [unwired: 1 in, 3 out]
      }
      event "Display On P1": Value Change {
        n1579 = event-data() -> ()  [unwired: 7 out]
        n1580 = Select(t="dim 100", s="Display On P1", f="dim 0") -> (s? t:f=w2234:string)
        n1581 = Concatenate Strings(w2234, "\r") -> (w2236:string)
        n1582 = VISA Write(VISA resource name=w2231, write buffer=w2236) -> ()  [unwired: 1 in, 3 out]
      }
      event "Retract Pump 3": Value Change {
        n1583 = event-data() -> ()  [unwired: 7 out]
        n1584 = local write "Retract Pump 3"(FALSE ("Retract Pump 3")) -> ()
        n1585 = case shown="True" "Retract Pump 3" {
          tunnel: w2238 -> [_ w2241]
          frame False {
          }
          frame True {
            n1586 = Number To Decimal String(number="Retract Rate (mL/m)") -> (decimal integer string=w2259:string)  [unwired: 1 in]
            n1587 = Concatenate Strings("wrate  " ("string"), w2259, " u/m" ("string"), "\r") -> (w2261:string)
            n1588 = VISA Write(VISA resource name=w2241, write buffer=w2261) -> (VISA resource name out=w2252:refnum<visa-resource-name>)  [unwired: 1 in, 2 out]
            n1589 = Number To Decimal String(number="Retract Vol 3 (uL)") -> (decimal integer string=w2254:string)  [unwired: 1 in]
            n1590 = Concatenate Strings("tvolume  " ("string"), w2254, " u" ("string"), "\r") -> (w2251:string)
            n1591 = VISA Write(VISA resource name=w2252, write buffer=w2251) -> (VISA resource name out=w2247:refnum<visa-resource-name>)  [unwired: 1 in, 2 out]
            n1592 = Concatenate Strings("cvolume" ("string"), "\r") -> (w2248:string)
            n1593 = VISA Write(VISA resource name=w2247, write buffer=w2248) -> (VISA resource name out=w2242:refnum<visa-resource-name>)  [unwired: 1 in, 2 out]
            n1594 = Concatenate Strings("wrun" ("string"), "\r") -> (w2243:string)
            n1595 = VISA Write(VISA resource name=w2242, write buffer=w2243) -> ()  [unwired: 1 in, 3 out]
          }
        }
      }
      event "Retract Pump 1": Value Change {
        n1596 = event-data() -> ()  [unwired: 7 out]
        n1597 = local write "Retract Pump 1"(FALSE ("Retract Pump 1")) -> ()
        n1598 = case shown="True" "Retract Pump 1" {
          tunnel: w2263 -> [_ w2268]
          frame False {
          }
          frame True {
            n1599 = local read "Retract Rate (mL/m)"() -> (w2266:dbl)
            n1600 = Number To Decimal String(number=w2266) -> (decimal integer string=w2284:string)  [unwired: 1 in]
            n1601 = Concatenate Strings("wrate  " ("string"), w2284, " u/m" ("string"), "\r") -> (w2286:string)
            n1602 = VISA Write(VISA resource name=w2268, write buffer=w2286) -> (VISA resource name out=w2278:refnum<visa-resource-name>)  [unwired: 1 in, 2 out]
            n1603 = Number To Decimal String(number="Retract Vol 1 (uL)") -> (decimal integer string=w2280:string)  [unwired: 1 in]
            n1604 = Concatenate Strings("tvolume  " ("string"), w2280, " u" ("string"), "\r") -> (w2277:string)
            n1605 = VISA Write(VISA resource name=w2278, write buffer=w2277) -> (VISA resource name out=w2274:refnum<visa-resource-name>)  [unwired: 1 in, 2 out]
            n1606 = Concatenate Strings("cvolume" ("string"), "\r") -> (w2275:string)
            n1607 = VISA Write(VISA resource name=w2274, write buffer=w2275) -> (VISA resource name out=w2269:refnum<visa-resource-name>)  [unwired: 1 in, 2 out]
            n1608 = Concatenate Strings("wrun" ("string"), "\r") -> (w2270:string)
            n1609 = VISA Write(VISA resource name=w2269, write buffer=w2270) -> ()  [unwired: 1 in, 3 out]
          }
        }
      }
      event "Flip Green Filter": Value Change {
        n1610 = event-data() -> ()  [unwired: 7 out]
        n1611 = Not(x="Flip Green Filter") -> (.not. x?=w2288:bool)
        n1612 = local write "Flip Green Filter"(w2288) -> ()
        n1613 = flat-sequence {
          tunnel: w2296 -> [w2301]
          tunnel: w2295 -> [w2300]
          tunnel: [w2298] -> w2293
          tunnel: [w2297] -> w2292
          tunnel: [w2303] -> w2291
          tunnel: w2293 -> [w2303]
          tunnel: [w2302] -> w2290
          tunnel: w2292 -> [w2302]
          tunnel: w2291 -> [w2307]
          tunnel: w2290 -> [w2306]
          tunnel: [w2305] -> w2294
          frame #0 {
            n1614 = xnode "Read/Write Control"("FPGA VI Reference In"=w2301, "error in"=w2300, "Green Filter Flipper"=TRUE) -> ("FPGA VI Reference Out"=w2298:T22, "error out"=w2297:errorcluster)
          }
          frame #1 {
            n1615 = Wait (ms)(milliseconds to wait=u32 100) -> ()  [unwired: 1 out]
          }
          frame #2 {
            n1616 = xnode "Read/Write Control"("FPGA VI Reference In"=w2307, "error in"=w2306, "Green Filter Flipper"=FALSE) -> ("error out"=w2305:errorcluster)  [unwired: 1 out]
          }
        }
      }
      event "Pump 1 contents", "Pump 3 contents": Value Change {
        n1617 = event-data() -> ()  [unwired: 7 out]
        n1618 = local read "Pump 1 contents"() -> (→"Pump 1 cont disp":string)
        n1619 = local read "Pump 3 contents"() -> (→"Pump 3 cont disp":string)
      }
      event "Reset Trap Pos. FB": Value Change {
        n1620 = event-data() -> ()  [unwired: 7 out]
        n1621 = xnode "Read/Write Control"("FPGA VI Reference In"=w2313, "error in"=w2312, "Trap Pos. FB Reset"="Reset Trap Pos. FB") -> ()  [unwired: 2 out]
      }
      event "Rem fb disp offset": Value Change {
        n1622 = event-data() -> ()  [unwired: 7 out]
        n1623 = local write "Rem fb disp offset"(FALSE ("Rem fb disp offset")) -> ()
        n1624 = local read "Mean T1 Position (nm)"() -> (w2315:dbl)
        n1625 = local read "FB Trap Pos Offset"() -> (w2316:dbl)
        n1626 = Subtract(x=w2316, y=w2315) -> (x-y=w2314:dbl)
        n1627 = local write "FB Trap Pos Offset"(w2314) -> ()
      }
      event "Threshold (nm)": Value Change {
        n1628 = event-data() -> ()  [unwired: 7 out]
        n1629 = flat-sequence {
          tunnel: w2320 -> [w2328]
          tunnel: w2319 -> [w2327]
          tunnel: [w2321] -> w2318
          tunnel: w2318 -> [w2334]
          frame #0 {
            n1630 = xnode "Read/Write Control"("FPGA VI Reference In"=w2328, "error in"=w2327) -> ("FPGA VI Reference Out"=w2324:T22, "error out"=w2323:errorcluster, "FPGA TTrig Thresh"=w2325:i64)
            n1631 = local read "Threshold stored (nm)"() -> (w2333:dbl)
            n1632 = local read "Threshold (nm)"() -> (w2321:dbl)
            n1633 = local read "AOM X Cal (nm/MHz)"() -> (w2331:dbl)
            n1634 = Subtract(x=w2321, y=w2333) -> (x-y=w2332:dbl)
            n1635 = Divide(x=w2332, y=w2331) -> (x/y=w2329:dbl)
            n1636 = call "IR AOM freq to word.vi"("Frequency In (MHz)"=w2329) -> ("Frequency Word Out (double)"=w2330:dbl)
            n1637 = To Quad Integer(1:w2330) -> (0:w2326:i64)
            n1638 = Add(x=w2325, y=w2326) -> (x+y=w2322:i64)
            n1639 = xnode "Read/Write Control"("FPGA VI Reference In"=w2324, "error in"=w2323, "FPGA TTrig Thresh"=w2322) -> ()  [unwired: 2 out]
          }
          frame #1 {
            "Threshold stored (nm)" <- w2334
          }
        }
      }
      event "FB Trig Integrate": Value Change {
        n1640 = event-data() -> ()  [unwired: 7 out]
        n1641 = local read "FB Trig Integrate"() -> (w2336:u32)
        n1642 = xnode "Read/Write Control"("FPGA VI Reference In"=w2338, "error in"=w2337, "FB Trig Integrate"=w2336) -> ("error out"=w2335:errorcluster)  [unwired: 1 out]
      }
      event "11": Value Change {
        n1643 = event-data() -> ()  [unwired: 7 out]
        n1644 = local read "11"() -> (w2339:bool)
        n1645 = case shown="True" w2339 {
          frame False {
          }
          frame True {
            n1646 = local read "Messages"() -> (w2341:string)
            n1647 = call "Update messages.vi"("Message to add"="You kicked it up to 11!", "Old message string"=w2341) -> ("New message string"=w2342:string)
            n1648 = call <vilib>:"Beep.vi"() -> ()  [unwired: 12 in]
            n1649 = local write "Messages"(w2342) -> ()
          }
        }
      }
      event "Trap Pos. FB ON": Value Change {
        n1650 = event-data() -> ()  [unwired: 7 out]
        n1651 = xnode "Read/Write Control"("FPGA VI Reference In"=w2345, "error in"=w2344, "Force feedback"="Trap Pos. FB ON") -> ()  [unwired: 2 out]
      }
      event "Remove Action Offset": Value Change {
        n1652 = event-data() -> ()  [unwired: 7 out]
        n1653 = local write "Remove Action Offset"(FALSE ("Remove Action Offset")) -> ()
        n1654 = local read "Trap Pos. FB Mult Factor"() -> (w2350:i64)
        n1655 = local read "Trap Pos FB Action"() -> (w2348:i64)
        n1656 = local read "Trap Pos. FB Offset Factor"() -> (w2346:i64)
        n1657 = Multiply(x=w2350, y=w2348) -> (x*y=w2349:i64)
        n1658 = Add(x=w2349, y=w2346) -> (x+y=w2347:i64)
        n1659 = local write "Trap Pos. FB Offset Factor"(w2347) -> ()
        n1660 = xnode "Read/Write Control"("FPGA VI Reference In"=w2353, "error in"=w2352, "Trap Pos. FB Offset Factor"=w2347) -> ()  [unwired: 2 out]
      }
      event "Remove Offset to factor": Value Change {
        n1661 = event-data() -> ()  [unwired: 7 out]
        n1662 = local write "Remove Offset to factor"(FALSE ("Remove Action Offset")) -> ()
        n1663 = local read "Trap Pos. FB Mult Factor"() -> (w2365:i64)
        n1664 = local read "Trap Pos FB Action"() -> (w2363:i64)
        n1665 = local read "Trap Pos. FB Offset Factor"() -> (w2362:i64)
        n1666 = Multiply(x=w2365, y=w2363) -> (x*y=w2364:i64)
        n1667 = local read "Trap Pos. FB Mult Factor"() -> (w2361:i64)
        n1668 = Add(x=w2364, y=w2362) -> (x+y=w2356:i64)
        n1669 = Multiply(x=32768, y="factor") -> (x*y=w2359:dbl)
        n1670 = Multiply(x=w2359, y=w2361) -> (x*y=w2360:dbl)
        n1671 = Subtract(x=w2356, y=w2360) -> (x-y=w2354:dbl)
        n1672 = To Quad Integer(1:w2354) -> (0:w2355:i64)
        n1673 = xnode "Read/Write Control"("FPGA VI Reference In"=w2368, "error in"=w2367, "Trap Pos. FB Offset Factor"=w2355) -> ()  [unwired: 2 out]
        n1674 = local write "Trap Pos. FB Offset Factor"(w2355) -> ()
      }
      event "Trap Pos. FB Range", "Trap Pos. FB Gains", "Trap Pos. FB Mult Factor", "Trap Pos. FB Offset Factor", "Trap Pos FB Negate Action", "Trap Pos FB Monitor\nT1 or T2", "Differential FB?", "Negate Diff?": Value Change {
        n1675 = event-data() -> ()  [unwired: 7 out]
        n1676 = local read "Negate Diff?"() -> (w2369:bool)
        n1677 = xnode "Read/Write Control"("FPGA VI Reference In"=w2379, "error in"=w2378, "Trap Pos. FB Range"="Trap Pos. FB Range", "Trap Pos. FB Gains"="Trap Pos. FB Gains", "Trap Pos. FB Mult Factor"="Trap Pos. FB Mult Factor", "Trap Pos. FB Offset Factor"="Trap Pos. FB Offset Factor", "Trap Pos FB Negate Action"="Trap Pos FB Negate Action", "Trap Pos FB Monitor T1 or T2"="Trap Pos FB Monitor\nT1 or T2", "AI1 X Scale"="Trap Pos. AI1 X Pre-scale", "Negate Diff?"=w2369, "Diff FB Measurement?"="Differential FB?") -> ()  [unwired: 2 out]
      }
      event "Trap Pos FB SP", "Trap Pos FB SP 2", "Use SP 2": Value Change {
        n1678 = event-data() -> ()  [unwired: 7 out]
        n1679 = Select(t="Trap Pos FB SP 2", s="Use SP 2", f="Trap Pos FB SP") -> (s? t:f=w2380:fxp<+/-,16,1>)
        n1680 = xnode "Read/Write Control"("FPGA VI Reference In"=w2385, "error in"=w2384, "Trap Pos. FB SP"=w2380) -> ()  [unwired: 2 out]
      }
      event "Offset SP2 from SP1": Value Change {
        n1681 = event-data() -> ()  [unwired: 7 out]
        n1682 = local read "Trap Pos FB SP"() -> (w2388:fxp<+/-,16,1>)
        n1683 = Add(x=w2388, y="SP2 Offset") -> (x+y=w2386:fxp<+/-,16,1>)
        n1684 = property on="Trap Pos FB SP 2" class="DigNum (strict)"("Val(Sgnl)"=w2386) -> ()  [unwired: 2 in, 2 out]
        n1685 = local write "Offset SP2 from SP1"(FALSE ("Offset SP2 from SP1")) -> ()
      }
      event "Set Reading to\nSetpoint": Value Change {
        # "This is the actual PID input signal"
        n1686 = event-data() -> ()  [unwired: 7 out]
        n1687 = local write "Set Reading to\nSetpoint"(FALSE ("Set SP to Reading")) -> ()
        n1688 = xnode "Read/Write Control"("FPGA VI Reference In"=w2394, "error in"=w2393) -> ("FPGA VI Reference Out"=w2392:T22, "error out"=w2391:errorcluster, "Trap Pos FB Int-Norm Signal"=w2390:fxp<+/-,16,1>)
        n1689 = local read "Differential FB?"() -> (w2395:bool)
        n1690 = case shown="False" w2395 {
          tunnel: [w2400 w2407] -> w2397
          tunnel: w2390 -> [w2398 w2407]
          frame False {
            n1691 = local read "Trap Pos FB Monitor\nT1 or T2"() -> (w2403:bool)
            n1692 = local read "Trap X AI1 (DMA)"() -> (w2406:T13)
            n1693 = Unbundle By Name(w2406) -> ("Set 1"=w2405:fxp<+/-,16,1>, "Set 2"=w2404:fxp<+/-,16,1>)
            n1694 = Select(t=w2405, s=w2403, f=w2404) -> (s? t:f=w2402:fxp<+/-,16,1>)
            n1695 = Not(x="Set SP Using...") -> (.not. x?=w2399:bool)
            n1696 = Select(t=w2398, s=w2399, f=w2402) -> (s? t:f=w2400:fxp<+/-,16,1>)
          }
          frame True {
          }
        }
        n1697 = xnode "Read/Write Control"("FPGA VI Reference In"=w2392, "error in"=w2391, "Trap Pos. FB SP"=w2397) -> ()  [unwired: 2 out]
        n1698 = local write "Trap Pos FB SP"(w2397) -> ()
      }
      event "Trap Pos. FB Out Scale 2^n": Value Change {
        n1699 = event-data() -> ()  [unwired: 7 out]
        n1700 = Scale By Power Of 2(n="Trap Pos. FB Out Scale 2^n", x=ext 1.0) -> (x*2^n=w2408:ext)
        n1701 = property on="Trap Pos. FB Mult Factor" class="DigNum (strict)"("Val(Sgnl)"=w2408) -> ()  [unwired: 2 in, 2 out]
      }
      event "Trap Pos FB Int Count": Value Change {
        n1702 = event-data() -> ()  [unwired: 7 out]
        n1703 = xnode "Read/Write Control"("FPGA VI Reference In"=w2413, "error in"=w2412, "Trap Pos FB Int Count"="Trap Pos FB Int Count") -> ()  [unwired: 2 out]
      }
      event "Trap pos": Value Change {
        n1704 = event-data() -> ()  [unwired: 7 out]
        n1705 = case shown="True" "Trap pos" {
          frame False {
            n1706 = property on="Trap Delta Graph" class="WFGraph (strict)"("Visible"=TRUE) -> ()  [unwired: 2 in, 2 out]
            n1707 = property on="Saved trap pos" class="WFGraph (strict)"("Visible"=FALSE) -> ()  [unwired: 2 in, 2 out]
          }
          frame True {
            n1708 = property on="Saved trap pos" class="WFGraph (strict)"("Visible"=TRUE) -> ()  [unwired: 2 in, 2 out]
            n1709 = property on="Trap Delta Graph" class="WFGraph (strict)"("Visible"=FALSE) -> ()  [unwired: 2 in, 2 out]
          }
        }
      }
      event "Save user params": Value Change {
        n1710 = event-data() -> ()  [unwired: 7 out]
        n1711 = local write "Save user params"(FALSE ("Save user\nparams")) -> ()
        n1712 = call "save control values.vi"("User"="User") -> ()  [unwired: 8 in, 1 out]
        n1713 = local read "Messages"() -> (w2425:string)
        n1714 = Concatenate Strings("User: ", "User", "\r", "Parameters saved.") -> (w2420:string)